vi "UHR-Fleezers Control (host) - 10.4.vi"() -> ()   [LabVIEW 2010] (continued)
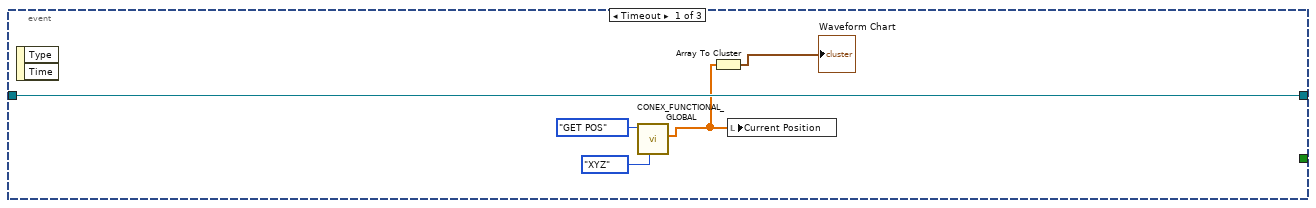
[diagram p2: hidden frame]
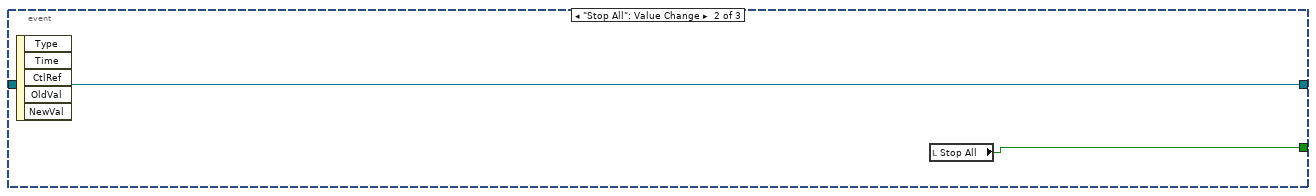
[diagram p3: hidden frame]
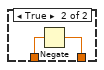
[diagram p4: hidden frame]
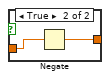
[diagram p5: hidden frame]
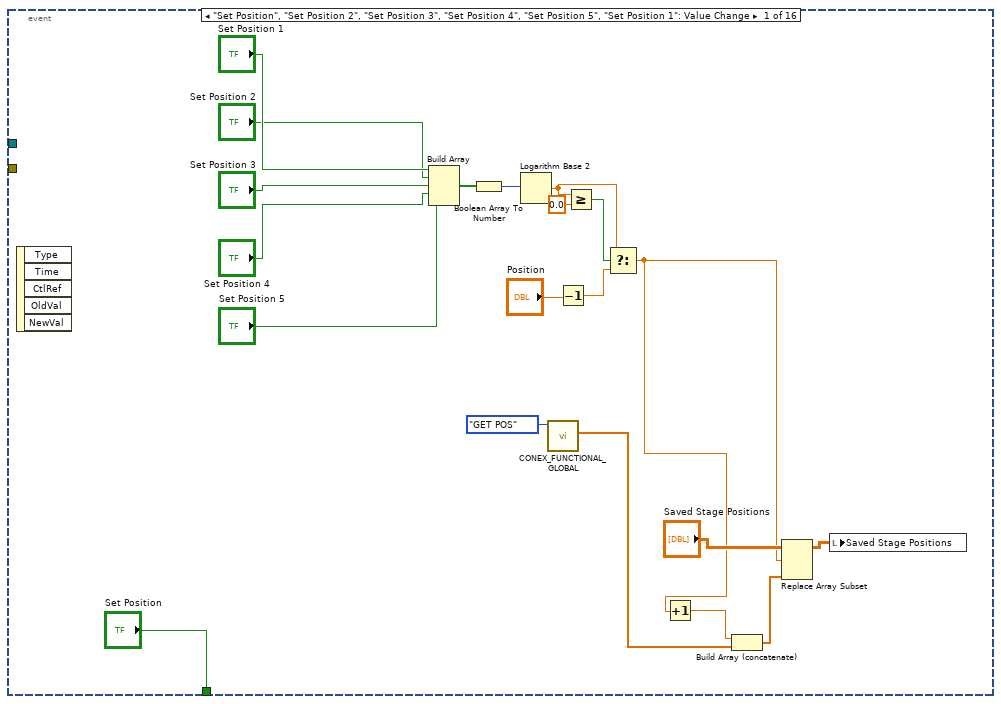
[diagram p6: hidden frame]
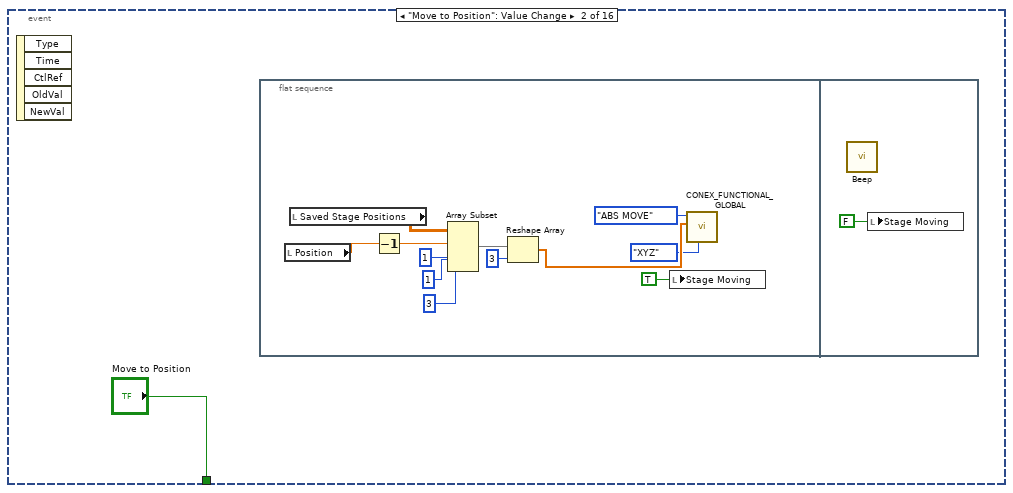
[diagram p7: hidden frame]
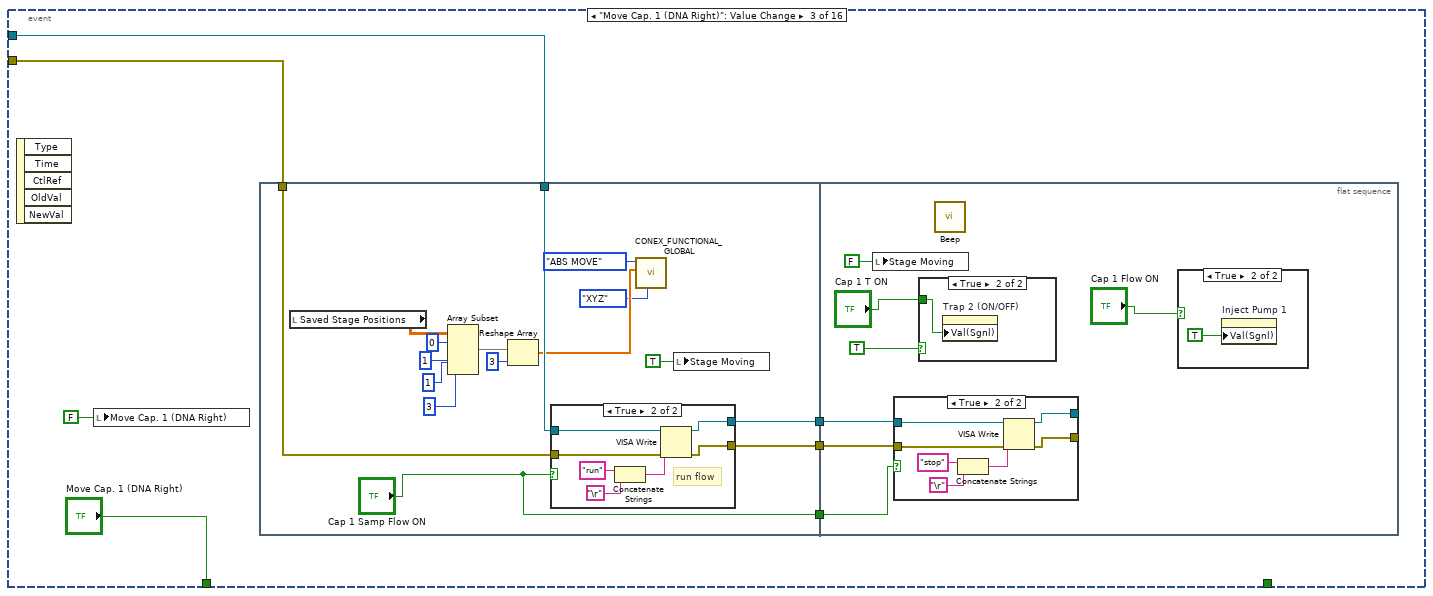
[diagram p8: hidden frame]
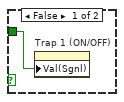
[diagram p12: hidden frame]
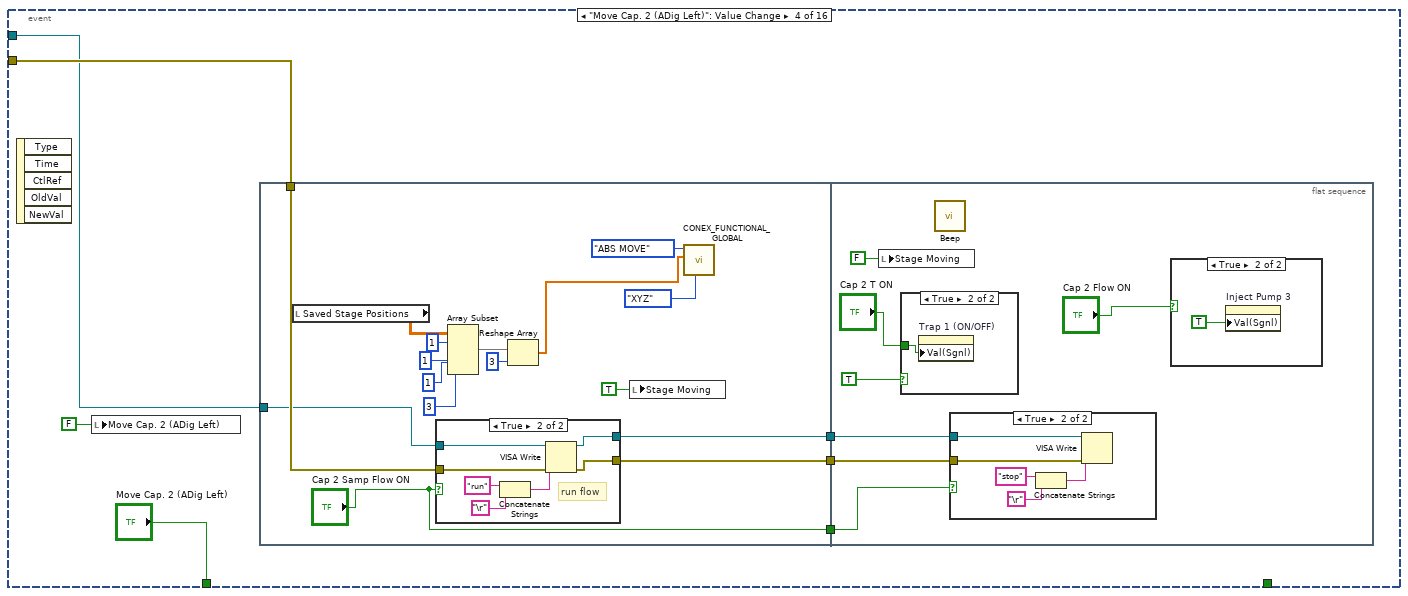
[diagram p13: hidden frame]
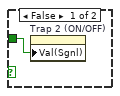
[diagram p17: hidden frame]
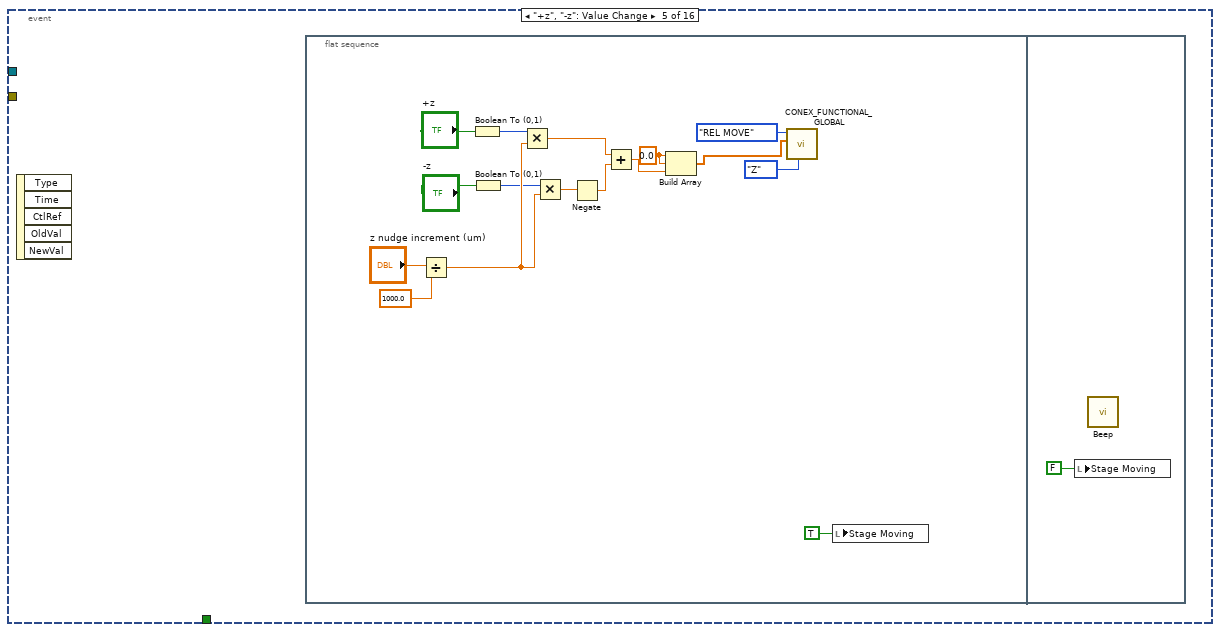
[diagram p18: hidden frame]
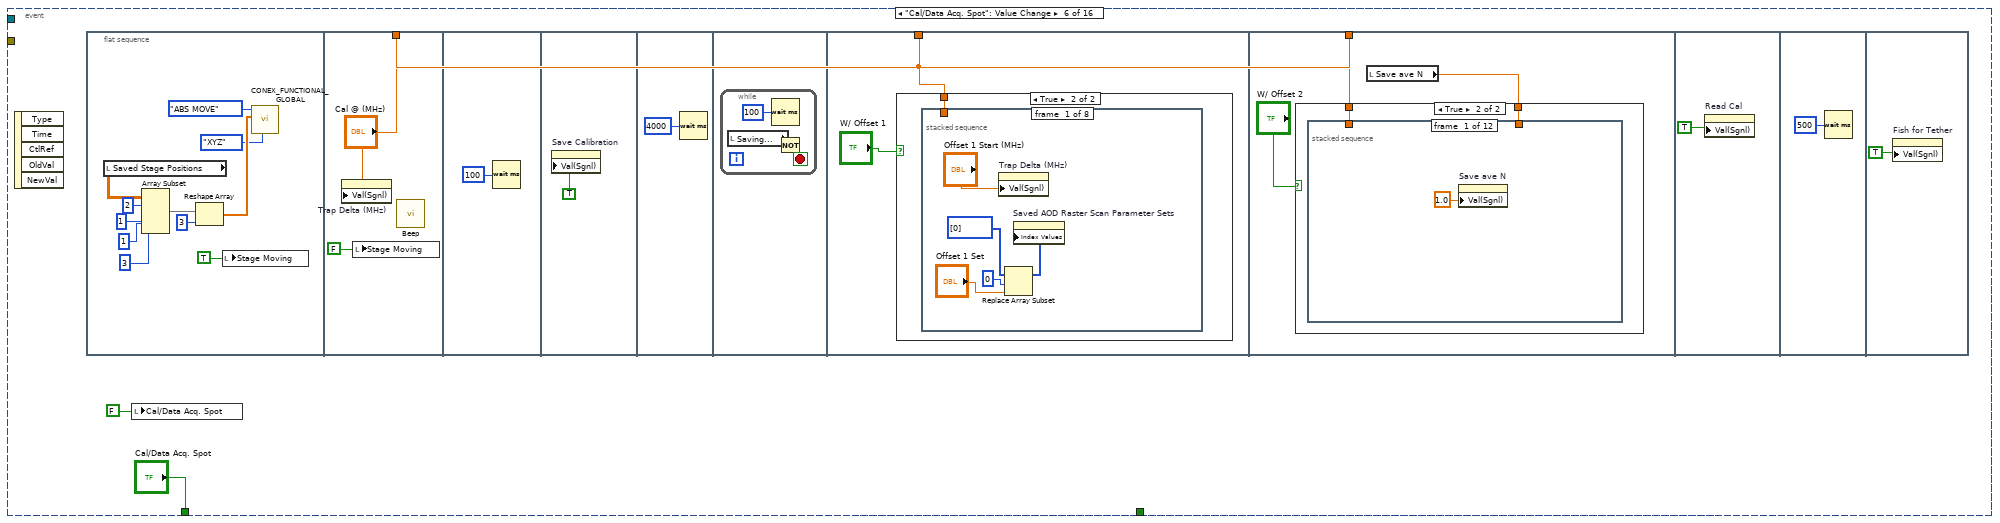
[diagram p19: hidden frame]
                  tunnel: w8360 -> [_ w8383]
                  frame False {
                  }
                  frame True {
                    n1983 = property on="AO2" class="Slide (strict)"("Val(Sgnl)"=w8383) -> ()  [unwired: 2 in, 2 out]
                  }
                }
                n1984 = case shown="True" w8352 {
                  tunnel: w8359 -> [_ w8384]
                  frame False {
                  }
                  frame True {
                    n1985 = property on="AO1" class="Slide (strict)"("Val(Sgnl)"=w8384) -> ()  [unwired: 2 in, 2 out]
                  }
                }
                n1986 = local write "Set Confocal Spot (X-Y)"(w8357) -> ()
                n1987 = local write "Set X Only"(w8357) -> ()
                n1988 = local write "Set Y Only"(w8357) -> ()
              }
            }
          }
          frame 3 {
            n1989 = local read "BD 2 Frequency 1 (MHz)"() -> (w8385:dbl)
            n1990 = local read "BD 1 Frequency 1 (MHz)"() -> (w8386:dbl)
            n1991 = local write "Manipulating Trap"(TRUE ("Manipulating Trap")) -> ()
            n1992 = local write "Coords"(T8 {"Horizontal"=0, "Vertical"=0} ("Coords")) -> ()
            n1993 = while {
              tunnel: w8391 -> [w8396]
              tunnel: w8389 -> [w8395]
              tunnel: w8387 -> [w8394]
              tunnel: w8386 -> [w8393]
              tunnel: w8385 -> [w8392]
              stop <- w8397 stop-if-true
              n1994 = event shown="[0] \"Pane\": Mouse Move" {
                selector: _ -> [_ _]
                dyn-events: _ -> [_ _]
                timeout: _ -> [_ _]
                tunnel: ["Force Manip Abort" w8461] -> w8397
                tunnel: w8396 -> [w8404 _]
                tunnel: w8395 -> [w8402 _]
                tunnel: w8394 -> [w8401 _]
                tunnel: w8393 -> [w8400 _]
                tunnel: w8392 -> [w8399 _]
                event Mouse Move {
                  n1995 = event-data() -> ("Time"=w8405:u32, "Coords"=w8406:T8)  [unwired: 3 out]
                  n1996 = Less?(x=w8405, y=w8404) -> (x < y?=w8403:bool)
                  n1997 = case "Makes sure old motion events prior to mouse click aren't used" shown="False" w8403 {
                    tunnel: w8406 -> [w8448 _]
                    tunnel: w8402 -> [w8449 _]
                    tunnel: w8401 -> [w8426 _]
                    tunnel: w8400 -> [w8422 _]
                    tunnel: w8399 -> [w8421 _]
                    frame False {
                      n1998 = Subtract(x=w8448, y=w8449) -> (x-y=w8447:T8)
                      "Coords" <- w8447
                      n1999 = local read "Y RF Frequency Limits (MHz)"() -> (w8407:T17)
                      n2000 = To Double Precision Float(number=w8447) -> (double precision float=w8446:cluster{"Horizontal":dbl, "Vertical":dbl})
                      n2001 = Multiply(x=cluster{"Horizontal":dbl, "Vertical":dbl} {"Horizontal"=-1.0, "Vertical"=1.0}, y="Manipulation Scaling") -> (x*y=w8442:cluster{"Horizontal":dbl, "Vertical":dbl})
                      n2002 = local read "X RF Frequency Limits (MHz)"() -> (w8408:T17)
                      n2003 = Multiply(x=w8446, y=w8442) -> (x*y=w8444:cluster{"Horizontal":dbl, "Vertical":dbl})
                      n2004 = Unbundle By Name(w8444) -> ("Horizontal"=w8439:dbl, "Vertical"=w8443:dbl)
                      n2005 = Unbundle By Name(w8407) -> ("Maximum"=w8410:dbl, "Minimum"=w8409:dbl)
                      n2006 = Boolean To (0,1)(Boolean="Manip. X?") -> (0, 1=w8437:i16)
                      n2007 = Boolean To (0,1)(Boolean="Manip. Y?") -> (0, 1=w8434:i16)
                      n2008 = local read "BD 1 Frequency 2 (MHz)"() -> (w8424:dbl)
                      n2009 = Multiply(x=w8443, y=w8434) -> (x*y=w8436:dbl)
                      n2010 = Multiply(x=w8437, y=w8439) -> (x*y=w8440:dbl)
                      n2011 = local read "BD 2 Frequency 2 (MHz)"() -> (w8423:dbl)
                      n2012 = Unbundle By Name(w8408) -> ("Maximum"=w8412:dbl, "Minimum"=w8411:dbl)
                      n2013 = Add(x=w8421, y=w8436) -> (x+y=w8414:dbl)
                      n2014 = Add(x=w8422, y=w8440) -> (x+y=w8416:dbl)
                      n2015 = In Range and Coerce(upper limit=w8412, x=w8416, lower limit=w8411) -> (coerced(x)=w8415:dbl)  [unwired: 1 out]
                      n2016 = In Range and Coerce(upper limit=w8410, x=w8414, lower limit=w8409) -> (coerced(x)=w8413:dbl)  [unwired: 1 out]
                      n2017 = Subtract(x=w8415, y=w8424) -> (x-y=w8433:dbl)
                      n2018 = Subtract(x=w8413, y=w8423) -> (x-y=w8432:dbl)
                      n2019 = Square(x=w8433) -> (x^2=w8431:dbl)
                      n2020 = Square(x=w8432) -> (x^2=w8430:dbl)
                      n2021 = Add(x=w8431, y=w8430) -> (x+y=w8429:dbl)
                      n2022 = Square Root(x=w8429) -> (sqrt(x)=w8425:dbl)
                      n2023 = In Range and Coerce(upper limit="Limit Max (MHz)", x=w8425, lower limit="Limit Min (MHz)") -> (In Range?=w8418:bool)  [unwired: 1 out]
                      n2024 = Not(x="Limits Enable") -> (.not. x?=w8417:bool)
                      n2025 = Or(x=w8418, y=w8417) -> (x .or. y?=w8419:bool)
                      n2026 = case shown="True" w8419 {
                        tunnel: w8426 -> [_ w8459]
                        tunnel: w8425 -> [_ w8450]
                        tunnel: w8415 -> [_ w8457]
                        tunnel: w8424 -> [_ w8456]
                        tunnel: w8413 -> [_ w8455]
                        tunnel: w8423 -> [_ w8454]
                        tunnel: w8408 -> [_ w8452]
                        tunnel: w8407 -> [_ w8451]
                        frame False {
                        }
                        frame True {
                          n2027 = local read "BD 1 Frequency 3 (MHz)"() -> (w8458:dbl)
                          n2028 = local read "BD 2 Frequency 3 (MHz)"() -> (w8453:dbl)
                          n2029 = local write "Trap Delta (MHz)"(w8450) -> ()
                          n2030 = property on="Initial delta (MHz)" class="DigNum (strict)"("Val(Sgnl)"=w8450) -> ()  [unwired: 2 in, 2 out]
                          n2031 = call "set RF board frequency - interlace.vi"("Board 2 Frequency Limits"=w8451, "Board 1 Frequency Limits"=w8452, "FPGA VI Reference In"=w8459, "Board 2 Frequency 3 (MHz)"=w8453, "Board 1 Frequency 3 (MHz)"=w8458, "Board 2 Frequency 2 (MHz)"=w8454, "Board 2 Frequency 1 (MHz)"=w8455, "Board 1 Frequency 2 (MHz)"=w8456, "Board 1 Frequency 1  (MHz)"=w8457) -> ()  [unwired: 1 in, 2 out]
                          n2032 = local write "BD 2 Frequency 1 (MHz)"(w8455) -> ()
                          n2033 = local write "BD 1 Frequency 1 (MHz)"(w8457) -> ()
                        }
                      }
                    }
                    frame True {
                    }
                  }
                }
                event Mouse Up {
                  n2034 = event-data() -> ("Button"=w8460:u16)  [unwired: 8 out]
                  n2035 = case shown="3" w8460 {
                    tunnel: [FALSE TRUE] -> w8461
                    frame 0, Default {
                    }
                    frame 3 {
                      n2036 = local write "Manipulating Trap"(FALSE ("Manipulating Trap")) -> ()
                    }
                  }
                }
              }
            }
          }
        }
      }
      event Mouse Move {
        n2037 = event-data() -> ()  [unwired: 6 out]
      }
    }
    n2038 = local read "Stop All"() -> (w8282:bool)
    n2039 = node-c288() -> ()  [unwired: 2 out]
  }
  n2040 = timed-loop "Oscillate AOD (debugging)" {
    tunnel: w18 -> [w8466]
    tunnel: [w8465] -> w68
    timing: w63 -> [_]
    timing-out: [_] -> w62
    stop <- w8465 stop-if-true
    n2041 = node-c288() -> ()  [unwired: 2 out]
    n2042 = event shown="[2] \"Stop All\": Value Change" {
      selector: _ -> [_ _ _]
      dyn-events: _ -> [_ _ _]
      timeout: _ -> [_ _ _]
      tunnel: w8466 -> [w8473 _ _]
      tunnel: [FALSE ("Stop All") _ w8742] -> w8465
      event "Oscillate Set 1", "Fish for Tether": Value Change {
        n2043 = event-data() -> ()  [unwired: 6 out]
        n2044 = local read "Oscillate Set 1"() -> (w8472:bool)
        n2045 = Or(x=w8472, y="Fish for Tether") -> (x .or. y?=w8470:bool)
        n2046 = case shown="True" w8470 {
          tunnel: w8473 -> [_ w8476]
          tunnel: "Fish for Tether" -> [_ w8475]
          frame False {
          }
          frame True {
            n2047 = case shown="False" w8475 {
              frame False {
              }
              frame True {
                n2048 = local write "Scan axis 2"(TRUE) -> ()
                n2049 = local write "Tether"(FALSE ("Tether")) -> ()
              }
            }
            n2050 = node-c288(i64 50 ("Period")) -> (w8478:T25)  [unwired: 3 out]
            n2051 = timed-loop "Oscillate AOD" {
              timing: w8478 -> [_]
              timing-out: [_] -> w8477
              tunnel: w8476 -> [w8488]
              tunnel: w8475 -> [w8487]
              i -> [w8490]
              stop <- w8486 stop-if-true
              n2052 = node-c288() -> (w8489:i64)  [unwired: 1 out]
              n2053 = flat-sequence {
                tunnel: w8490 -> [w8517]
                tunnel: w8489 -> [w8516]
                tunnel: w8488 -> [w8497]
                tunnel: w8487 -> [w8500]
                tunnel: [w8500] -> w8485
                tunnel: [w8499] -> w8484
                tunnel: [w8496] -> w8483
                tunnel: [w8493] -> w8481
                tunnel: w8485 -> [w8553]
                tunnel: w8484 -> [w8551]
                tunnel: w8483 -> [w8550]
                tunnel: [w8549] -> w8482
                tunnel: w8481 -> [w8548]
                tunnel: [w8617] -> w8486
                tunnel: w8482 -> [w8615]
                frame #0 {
                  n2054 = Divide(x=w8516, y=i64 1000) -> (x/y=w8511:dbl)
                  n2055 = Multiply(x=w8511, y=w8517) -> (x*y=w8513:dbl)
                  n2056 = Multiply(x="Osc. freq. (Hz)", y=6.283185307179586) -> (x*y=w8514:dbl)
                  n2057 = Multiply(x=w8514, y=w8513) -> (x*y=w8495:dbl)
                  n2058 = local read "BD 1 Frequency 2 (MHz)"() -> (w8498:dbl)
                  n2059 = local read "BD 1 Frequency 1 (MHz)"() -> (w8491:dbl)
                  n2060 = case shown="False" w8500 {
                    tunnel: w8495 -> [w8523 w8529]
                    tunnel: w8498 -> [_ w8540]
                    tunnel: [w8520 w8535] -> w8501
                    tunnel: [FALSE w8532] -> w8496
                    tunnel: [0.0 w8525] -> w8493
                    tunnel: w8491 -> [_ w8524]
                    frame False {
                      n2061 = Sine(x=w8523) -> (sin(x)=w8521:dbl)
                      n2062 = Multiply(x=w8521, y="Osc. amp. (MHz)") -> (x*y=w8520:dbl)
                    }
                    frame True {
                      n2063 = Cosine(x=w8529) -> (cos(x)=w8543:dbl)
                      n2064 = Subtract(x=w8540, y=w8524) -> (x-y=w8539:dbl)
                      n2065 = Decrement(x=w8543) -> (x-1=w8542:dbl)
                      n2066 = Subtract(x=w8539, y="Closest Delta (MHz)") -> (x-y=w8536:dbl)
                      n2067 = Divide(x=w8542, y=-2.0) -> (x/y=w8537:dbl)
                      n2068 = Multiply(x=w8537, y=w8536) -> (x*y=w8535:dbl)
                      n2069 = local read "Vec Mean of T1 T2"() -> (w8531:dbl[])
                      n2070 = Greater?(x=w8531, y="Stop F (pN)") -> (0:w8533:bool[])
                      n2071 = Or Array Elements(Boolean array=w8533) -> (logical OR=w8532:bool)
                      n2072 = Divide(x=w8529, y=6.283185307179586) -> (x/y=w8528:dbl)
                      n2073 = Round Toward +Infinity(x=w8528) -> (ceil(x): smallest int >= x=w8525:dbl)
                      "Attempts" <- w8525
                      n2074 = Greater?(x=w8525, y="Attempt Limit") -> (0:w8527:bool)
                      n2075 = case shown="True" w8527 {
                        frame False {
                        }
                        frame True {
                          n2076 = local write "Fish for Tether"(FALSE ("Fish for Tether")) -> ()
                          n2077 = call <vilib>:"Beep.vi"() -> ()  [unwired: 3 in, 9 out]
                          n2078 = local read "Messages"() -> (w8545:string)
                          n2079 = call "Update messages.vi"("Message to add"="Tether fishing timeout." ("Messages"), "Old message string"=w8545) -> ("New message string"=→"Messages":string)
                        }
                      }
                    }
                  }
                  n2080 = local read "BD 2 Frequency 1 (MHz)"() -> (w8502:dbl)
                  n2081 = Select(t=w8491, s="Scan axis 2", f=w8502) -> (s? t:f=w8505:dbl)
                  n2082 = Add(x=w8501, y=w8505) -> (x+y=w8499:dbl)
                  n2083 = Select(t=w8499, s="Scan axis 2", f=w8491) -> (s? t:f=w8492:dbl)
                  n2084 = Select(t=w8502, s="Scan axis 2", f=w8499) -> (s? t:f=w8507:dbl)
                  n2085 = local read "Y RF Frequency Limits (MHz)"() -> (w8503:T17)
                  n2086 = local read "X RF Frequency Limits (MHz)"() -> (w8504:T17)
                  n2087 = local read "BD 1 Frequency 3 (MHz)"() -> (w8510:dbl)
                  n2088 = local read "BD 2 Frequency 2 (MHz)"() -> (w8509:dbl)
                  n2089 = local read "BD 2 Frequency 3 (MHz)"() -> (w8508:dbl)
                  n2090 = call "set RF board frequency - interlace.vi"("Board 2 Frequency Limits"=w8503, "Board 1 Frequency Limits"=w8504, "FPGA VI Reference In"=w8497, "Board 2 Frequency 3 (MHz)"=w8508, "Board 1 Frequency 3 (MHz)"=w8510, "Board 2 Frequency 2 (MHz)"=w8509, "Board 2 Frequency 1 (MHz)"=w8507, "Board 1 Frequency 2 (MHz)"=w8498, "Board 1 Frequency 1  (MHz)"=w8492) -> ()  [unwired: 1 in, 2 out]
                }
                frame #1 {
                  n2091 = And(x=w8553, y=w8550) -> (x .and. y?=w8552:bool)
                  n2092 = case "Only if were fishing and now formed tether" shown="False" w8552 {
                    tunnel: w8551 -> [w8555 w8567]
                    tunnel: [w8554 w8566] -> w8549
                    tunnel: w8548 -> [_ w8562]
                    frame False {
                      n2093 = local read "Fish for Tether"() -> (w8554:bool)
                      n2094 = case shown="False" w8554 {
                        tunnel: w8555 -> [_ _]
                        frame False {
                        }
                        frame True {
                        }
                      }
                    }
                    frame True {
                      w8566 = FALSE ("Fish for Tether")
                      n2095 = call <vilib>:"Beep.vi"() -> ()  [unwired: 3 in, 9 out]
                      n2096 = Number To Decimal String(number=w8562, width (-)=i16 1) -> (decimal integer string=w8560:string)
                      n2097 = case shown="\"1\", Default" "Then..." {
                        selector: "Then..." -> [_ w8570]
                        tunnel: w8567 -> [w8569 _]
                        frame "1", Default {
                          n2098 = property on="BD 1 Frequency 1 (MHz)" class="DigNum (strict)"("Val(Sgnl)"=w8569) -> ()  [unwired: 2 in, 2 out]
                        }
                        frame "2", "3", "4", "5", "6" {
                          n2099 = flat-sequence {
                            tunnel: w8570 -> [w8572]
                            frame #0 {
                              n2100 = property on="Trap Delta (MHz)" class="DigNum (strict)"("Val(Sgnl)"="Move to Delta 1 (MHz)") -> ()  [unwired: 2 in, 2 out]
                            }
                            frame #1 {
                              n2101 = case shown="\"5\", \"6\"" w8572 {
                                selector: w8572 -> [w8575 w8585 _]
                                frame "3", "4" {
                                n2102 = flat-sequence {
                                tunnel: w8575 -> [w8576]
                                tunnel: [w8576] -> w8573
                                tunnel: [w8578] -> w8574
                                tunnel: w8573 -> [w8578]
                                tunnel: w8574 -> [w8582]
                                frame #0 {
                                n2103 = property on="Green Laser ON/Interlacing" class="Bool (strict)"("Val(Sgnl)"=TRUE ("Value (Signaling)")) -> ()  [unwired: 2 in, 2 out]
                                }
                                frame #1 {
                                n2104 = Multiply(x="Wait Before Save (s)", y=u32 1000 ("x")) -> (x*y=w8580:u32)
                                n2105 = Wait (ms)(milliseconds to wait=w8580) -> ()  [unwired: 1 out]
                                }
                                frame #2 {
                                n2106 = property on="Start Saving" class="Bool (strict)"("Value"=TRUE ("Start Saving")) -> ()  [unwired: 2 in, 2 out]
                                n2107 = case shown="\"4\"" w8582 {
                                frame Default {
                                }
                                frame "4" {
                                n2108 = property on="Fl. Triggered..." class="Bool (strict)"("Val(Sgnl)"=TRUE ("Value (Signaling)")) -> ()  [unwired: 2 in, 2 out]
                                }
                                }
                                }
                                }
                                }
                                frame "5", "6" {
                                n2109 = stacked-sequence {
                                tunnel: w8585 -> [_ _ _ _ _ _ _ _ w8602 _ _]
                                frame #0 {
                                n2110 = Replace Array Subset(array=u32[] [0] ("Index Values"), new element="Raster Set Upon Tether", index=0) -> (w8586:u32[])
                                n2111 = property on="Saved AOD Raster Scan Parameter Sets" class="Arr (strict)"("Index Values"=w8586) -> ()  [unwired: 2 in, 2 out]
                                }
                                frame #1 {
                                n2112 = Wait (ms)(milliseconds to wait=u32 500) -> ()  [unwired: 1 out]
                                }
                                frame #2 {
                                n2113 = property on="Load parameters" class="Bool (strict)"("Val(Sgnl)"=TRUE ("Value (Signaling)")) -> ()  [unwired: 2 in, 2 out]
                                }
                                frame #3 {
                                n2114 = Wait (ms)(milliseconds to wait=u32 500) -> ()  [unwired: 1 out]
                                }
                                frame #4 {
                                n2115 = property on="Trap Raster Scan" class="Bool (strict)"("Val(Sgnl)"=TRUE ("Value (Signaling)")) -> ()  [unwired: 2 in, 2 out]
                                }
                                frame #5 {
                                n2116 = Wait (ms)(milliseconds to wait=u32 2000) -> ()  [unwired: 1 out]
                                }
                                frame #6 {
                                n2117 = while {
                                stop <- w8597 stop-if-true
                                n2118 = local read "Raster Scanning..."() -> (w8596:bool)
                                n2119 = local read "Saving..."() -> (w8599:bool)
                                n2120 = Wait (ms)(milliseconds to wait=u32 100) -> ()  [unwired: 1 out]
                                n2121 = Not(x=w8599) -> (.not. x?=w8598:bool)
                                n2122 = Not(x=w8596) -> (.not. x?=w8595:bool)
                                n2123 = And(x=w8598, y=w8595) -> (x .and. y?=w8597:bool)
                                }
                                }
                                frame #7 {
                                n2124 = property on="Trap Delta (MHz)" class="DigNum (strict)"("Val(Sgnl)"="Move to Delta 2 (MHz)") -> ()  [unwired: 2 in, 2 out]
                                }
                                frame #8 {
                                n2125 = local read "Tether"() -> (w8603:bool)
                                n2126 = case shown="True" w8603 {
                                tunnel: w8602 -> [_ w8604]
                                frame False {
                                }
                                frame True {
                                n2127 = flat-sequence {
                                tunnel: w8604 -> [w8606]
                                frame #0 {
                                n2128 = Wait (ms)(milliseconds to wait=u32 500) -> ()  [unwired: 1 out]
                                }
                                frame #1 {
                                n2129 = case shown="\"6\"" w8606 {
                                frame Default {
                                }
                                frame "6" {
                                n2130 = property on="Green Laser ON/Interlacing" class="Bool (strict)"("Val(Sgnl)"=TRUE ("Green Laser ON/Interlacing")) -> ()  [unwired: 2 in, 2 out]
                                }
                                }
                                }
                                frame #2 {
                                n2131 = Wait (ms)(milliseconds to wait=u32 500) -> ()  [unwired: 1 out]
                                }
                                frame #3 {
                                n2132 = local write "Start Saving"("Save at end (5, 6)") -> ()
                                }
                                }
                                }
                                }
                                }
                                frame #9 {
                                n2133 = local read "Bead Sep. Int. Time (s)"() -> (w8612:dbl)
                                n2134 = Multiply(x=w8612, y=1000.0) -> (x*y=w8611:dbl)
                                n2135 = Wait (ms)(milliseconds to wait=w8611) -> ()  [unwired: 1 out]
                                }
                                frame #10 {
                                n2136 = property on="Rescale on Mean" class="Bool (strict)"("Val(Sgnl)"=TRUE ("Value (Signaling)")) -> ()  [unwired: 2 in, 2 out]
                                }
                                }
                                }
                                frame "2", Default {
                                }
                              }
                            }
                          }
                        }
                      }
                      n2137 = Concatenate Strings("Formed tether in ", w8560, " attempt(s)." ("string")) -> (w8557:string)
                      n2138 = local read "Messages"() -> (w8564:string)
                      n2139 = local write "Fish for Tether"(w8566) -> ()
                      n2140 = call "Update messages.vi"("Message to add"=w8557, "Old message string"=w8564) -> ("New message string"=w8563:string)
                      n2141 = local write "Messages"(w8563) -> ()
                      n2142 = Get Date/Time In Seconds() -> (seconds since 1Jan1904=→"Time tether formed":timestamp)
                      "Tether" <- "Tether Alarm?"
                    }
                  }
                }
                frame #2 {
                  n2143 = local read "Oscillate Set 1"() -> (w8616:bool)
                  n2144 = local read "Stop All"() -> (w8618:bool)
                  n2145 = Not Or(1:w8615, 2:w8616) -> (0:w8614:bool)
                  n2146 = Compound Arithmetic op=OR(w8618, w8614) -> (w8617:bool)
                }
              }
              n2147 = node-c288() -> ()  [unwired: 2 out]
            }
            n2148 = node-c288(w8477) -> ()  [unwired: 1 out]
          }
        }
      }
      event "Fl. Triggered...": Value Change {
        n2149 = event-data() -> ()  [unwired: 7 out]
        n2150 = case shown="True" "Fl. Triggered..." {
          frame False {
          }
          frame True {
            n2151 = node-c288() -> (w8630:T25)  [unwired: 4 out]
            n2152 = timed-loop {
              timing: w8630 -> [_]
              timing-out: [_] -> w8629
              tunnel: "Action" -> [w8634]
              shift-right: [w8631] -> _
              shift-left: u8 255 -> [w8633]
              stop <- w8635 stop-if-true
              n2153 = node-c288() -> ()  [unwired: 2 out]
              n2154 = flat-sequence {
                tunnel: w8634 -> [w8647]
                tunnel: w8633 -> [w8644]
                tunnel: [w8643] -> w8632
                tunnel: [w8733] -> w8635
                tunnel: w8632 -> [w8732]
                tunnel: [w8732] -> w8631
                frame #0 {
                  n2155 = local read "Delta Fl. 2"() -> (w8638:dbl)
                  n2156 = local read "Delta Fl. 1"() -> (w8639:dbl)
                  n2157 = Select(t=w8639, s="APD to Watch", f=w8638) -> (s? t:f=w8637:dbl)
                  n2158 = Multiply(x="Fl. Delta Thresh. (kHz)", y=1000.0) -> (x*y=w8646:dbl)
                  n2159 = Greater?(x=w8637, y=w8646) -> (0:w8641:bool)
                  n2160 = Or(x="Force Yank", y=w8641) -> (x .or. y?=w8642:bool)
                  n2161 = case shown="True" w8642 {
                    tunnel: w8647 -> [_ w8657]
                    tunnel: w8644 -> [w8649 w8653]
                    tunnel: [w8649 w8650] -> w8643
                    frame False {
                    }
                    frame True {
                      n2162 = flat-sequence {
                        tunnel: w8654 -> [w8663]
                        tunnel: [w8663] -> w8658
                        tunnel: w8657 -> [w8662]
                        tunnel: [w8662] -> w8656
                        tunnel: [w8661] -> w8655
                        tunnel: w8653 -> [w8660]
                        tunnel: [w8659] -> w8652
                        tunnel: w8658 -> [w8688]
                        tunnel: w8656 -> [w8687]
                        tunnel: w8655 -> [w8686]
                        tunnel: w8652 -> [w8685]
                        tunnel: [w8685] -> w8651
                        tunnel: w8651 -> [w8730]
                        tunnel: [w8730] -> w8650
                        frame #0 {
                          n2163 = call <vilib>:"Beep.vi"() -> ()  [unwired: 3 in, 9 out]
                          n2164 = local write "Waiting"(FALSE ("Waiting")) -> ()
                          n2165 = Increment(x=w8660) -> (x+1=w8659:u8)
                          n2166 = case shown="\"Yank\"" w8662 {
                            tunnel: w8659 -> [_ _ w8669]
                            frame "Image" {
                              n2167 = property on="Confocal Image" class="Bool (strict)"("Val(Sgnl)"=TRUE ("Value (Signaling)")) -> ()  [unwired: 2 in, 2 out]
                            }
                            frame "Alarm", Default {
                            }
                            frame "Yank" {
                              n2168 = flat-sequence {
                                tunnel: w8669 -> [w8672]
                                tunnel: [w8671] -> w8668
                                tunnel: ["N Array El"] -> w8667
                                tunnel: w8668 -> [w8682]
                                tunnel: w8667 -> [w8678]
                                frame #0 {
                                n2169 = Multiply(x="Yank Delay (s)", y=1000.0) -> (x*y=w8675:dbl)
                                n2170 = Quotient & Remainder(x=w8672, y="N Array El") -> (x-y*floor(x/y)=w8671:u8)  [unwired: 1 out]
                                n2171 = Wait (ms)(milliseconds to wait=w8675) -> ()  [unwired: 1 out]
                                }
                                frame #1 {
                                n2172 = Random Number (0-1)() -> (number: 0 to 1=w8679:dbl)
                                n2173 = Multiply(x=w8678, y=w8679) -> (x*y=w8677:dbl)
                                n2174 = Round Toward -Infinity(1:w8677) -> (0:w8676:dbl)
                                n2175 = Select(t=w8676, s="Random Choice", f=w8682) -> (s? t:f=w8680:dbl)
                                n2176 = Index Array(array="Yank to Delta Array (MHz)", index=w8680) -> (element=w8683:dbl)
                                n2177 = property on="Trap Delta (MHz)" class="DigNum (strict)"("Val(Sgnl)"=w8683) -> ()  [unwired: 2 in, 2 out]
                                }
                              }
                            }
                          }
                          n2178 = local read "Time (s)"() -> (w8661:dbl)
                          "Fl. High" <- TRUE ("Yanking")
                        }
                        frame #1 {
                          n2179 = node-c288() -> (w8690:T25)  [unwired: 4 out]
                          n2180 = timed-loop {
                            timing: w8690 -> [_]
                            timing-out: [_] -> w8689
                            tunnel: w8688 -> [w8706]
                            tunnel: w8687 -> [w8704]
                            tunnel: w8686 -> [w8703]
                            stop <- w8705 stop-if-true
                            n2181 = node-c288() -> ()  [unwired: 2 out]
                            n2182 = local read "Fl. Delta Thresh. (kHz)"() -> (w8698:dbl)
                            n2183 = local read "Fl. Triggered..."() -> (w8707:bool)
                            n2184 = local read "Delta Fl. 1"() -> (w8694:dbl)
                            n2185 = local read "Delta Fl. 2"() -> (w8692:dbl)
                            n2186 = local read "Stop All"() -> (w8701:bool)
                            n2187 = local read "APD to Watch"() -> (w8693:bool)
                            n2188 = Select(t=w8694, s=w8693, f=w8692) -> (s? t:f=w8691:dbl)
                            n2189 = Not(x=w8707) -> (.not. x?=w8702:bool)
                            n2190 = Multiply(x=w8698, y=1000.0) -> (x*y=w8697:dbl)
                            n2191 = Negate(x=w8697) -> (-x=w8696:dbl)
                            n2192 = Less?(x=w8691, y=w8696) -> (x < y?=w8700:bool)
                            n2193 = Compound Arithmetic op=OR(w8700, w8701, w8702, "Force Reset") -> (w8705:bool)
                            n2194 = case shown="True" w8705 {
                              tunnel: w8706 -> [_ w8718]
                              tunnel: w8704 -> [_ w8717]
                              tunnel: w8703 -> [_ w8715]
                              frame False {
                              }
                              frame True {
                                n2195 = case shown="\"Yank\"" w8717 {
                                tunnel: w8718 -> [_ w8719]
                                frame "Image", Default {
                                }
                                frame "Yank" {
                                n2196 = flat-sequence {
                                tunnel: [w8724] -> w8720
                                tunnel: w8719 -> [w8724]
                                tunnel: w8720 -> [w8725]
                                frame #0 {
                                n2197 = local read "Yank Delay (s)"() -> (w8723:dbl)
                                n2198 = Multiply(x=w8723, y=1000.0) -> (x*y=w8721:dbl)
                                n2199 = Wait (ms)(milliseconds to wait=w8721) -> ()  [unwired: 1 out]
                                }
                                frame #1 {
                                n2200 = property on="Trap Delta (MHz)" class="DigNum (strict)"("Val(Sgnl)"=w8725) -> ()  [unwired: 2 in, 2 out]
                                }
                                }
                                }
                                }
                                n2201 = local read "Time (s)"() -> (w8716:dbl)
                                n2202 = Subtract(x=w8716, y=w8715) -> (x-y=w8712:dbl)
                                "Duration (s)" <- w8712
                                n2203 = Number To Decimal String(number=w8712, width (-)=i16 0) -> (decimal integer string=w8710:string)
                                n2204 = Concatenate Strings(w8710, " s fluorescence event." ("string")) -> (w8708:string)
                                n2205 = local read "Messages"() -> (w8714:string)
                                n2206 = call "Update messages.vi"("Message to add"=w8708, "Old message string"=w8714) -> ("New message string"=w8713:string)
                                n2207 = call <vilib>:"Beep.vi"() -> ()  [unwired: 3 in, 9 out]
                                n2208 = local write "Messages"(w8713) -> ()
                              }
                            }
                            n2209 = node-c288() -> ()  [unwired: 2 out]
                          }
                          n2210 = node-c288(w8689) -> ()  [unwired: 1 out]
                        }
                        frame #2 {
                          n2211 = local write "Fl. High"(FALSE ("Yanking")) -> ()
                        }
                      }
                      n2212 = local read "Trap Delta (MHz)"() -> (w8654:dbl)
                    }
                  }
                }
                frame #1 {
                  n2213 = local read "Stop All"() -> (w8736:bool)
                  n2214 = local read "Fl. Triggered..."() -> (w8734:bool)
                  n2215 = Not(x=w8734) -> (.not. x?=w8735:bool)
                  n2216 = Or(x=w8735, y=w8736) -> (x .or. y?=w8733:bool)
                  n2217 = Not(x=w8733) -> (.not. x?=→"Waiting":bool)
                }
              }
              n2218 = node-c288() -> ()  [unwired: 2 out]
            }
            n2219 = node-c288(w8629) -> ()  [unwired: 1 out]
          }
        }
      }
      event "Stop All": Value Change {
        n2220 = event-data() -> ()  [unwired: 7 out]
        n2221 = local read "Stop All"() -> (w8742:bool)
      }
    }
    n2222 = node-c288() -> ()  [unwired: 2 out]
  }
  n2223 = node-c288(w16) -> ()  [unwired: 1 out]
  n2224 = call-poly <vilib>:"Close Input Device.vi"("device ID"=w1) -> ()  [unwired: 9 in, 1 out]
  n2225 = call <vilib>:"IMAQ Stop.vi"("error in (no error)"=w3, "IMAQ Session In"=w5) -> ("error out"=w7:errorcluster, "IMAQ Session Out"=w6:refnum<k11>)  [unwired: 8 in]
  n2226 = call "IMAQ Dispose"("Image"=w4) -> ()  [unwired: 5 in, 1 out]
  n2227 = call <vilib>:"IMAQ Close.vi"("error in (no error)"=w7, "IMAQ Session In"=w6) -> ()  [unwired: 9 in, 1 out]
  n2228 = node-c288(w64) -> ()  [unwired: 1 out]
  n2229 = node-c288(w56) -> ()  [unwired: 1 out]
  n2230 = node-c288(w66) -> ()  [unwired: 1 out]
  n2231 = node-c288(w62) -> ()  [unwired: 1 out]
  n2232 = node-c288(w161) -> ()  [unwired: 1 out]
  n2233 = flat-sequence {
    tunnel: w256 -> [w8746]
    tunnel: w258 -> [w8747]
    tunnel: [w8745] -> w237
    tunnel: [w8744] -> w236
    tunnel: w218 -> [_]
    tunnel: w216 -> [_]
    tunnel: w169 -> [_]
    tunnel: w68 -> [_]
    tunnel: w237 -> [w8807]
    tunnel: w236 -> [w8808]
    frame #0 {
      w8743 = FALSE ("AI to FIFO")
      n2234 = xnode "Read/Write Control"("FPGA VI Reference In"=w8747, "error in"=w8746, "AI to FIFO"=w8743, "APD to FIFO"=w8743) -> ("FPGA VI Reference Out"=w8745:T20, "error out"=w8744:errorcluster)
    }
    frame #1 {
      n2235 = xnode "Close FPGA VI Reference"("FPGA VI Reference In"=w8807, "error in"=w8808) -> ("error out"=→"error out":errorcluster)
    }
  }
